vi "front_panel_v1.vi"() -> ()   [LabVIEW 2021]
uses:
  <vilib>/Platform/TimedLoop/XDataNode/timing_clust.ctl
  <vilib>/Platform/TimedLoop/XDataNode/nitl_modes.ctl
  <vilib>/Platform/TimedLoop/XDataNode/wakeup.ctl
  Global 1.vi
  <vilib>/platform/TimedLoop/XDataNode/XDataNode.xnode
  <vilib>/Platform/TimedLoop/XDataNode/XDNodeRunTimeDep.lvlib
panel:
  in  "Glove Address":string
  in  "Robotic Hand Address":string="192.168.4.93"
  out "Thumb 3":dbl
  out "Index Finger 2":dbl
  out "Middle Finger3":dbl
  out "Ring Finger 3":dbl
  out "Pinky Finger 2":dbl
  out "Simulation Connected":bool
  in  "Stop":bool
  in  "Stop Testing 2":bool
  out "Hand Status":bool
  out "Glove Status":bool
  in  "Stop Execution":bool
  in  "?":T1(tab)=enum."General Testing"
  out "Pinky Calibration":bool
  out "Ring Finger Calibration":bool
  out "Middle Finger Calibration":bool
  out "Index Calibration":bool
  out "Thumb Calibration":bool
  out "Glove SIgnal":dbl[](array[numeric])
  out "Waveform Chart":T2(graph)
  in  "Stop Testing":bool
  out "Output From Knob":string
  in  "Pinky":dbl(slide)
  in  "Ring Finger":dbl(slide)
  in  "Index":dbl(slide)
  in  "Middle Finger":dbl(slide)=85.0
  in  "Thumb":dbl(slide)=90.0
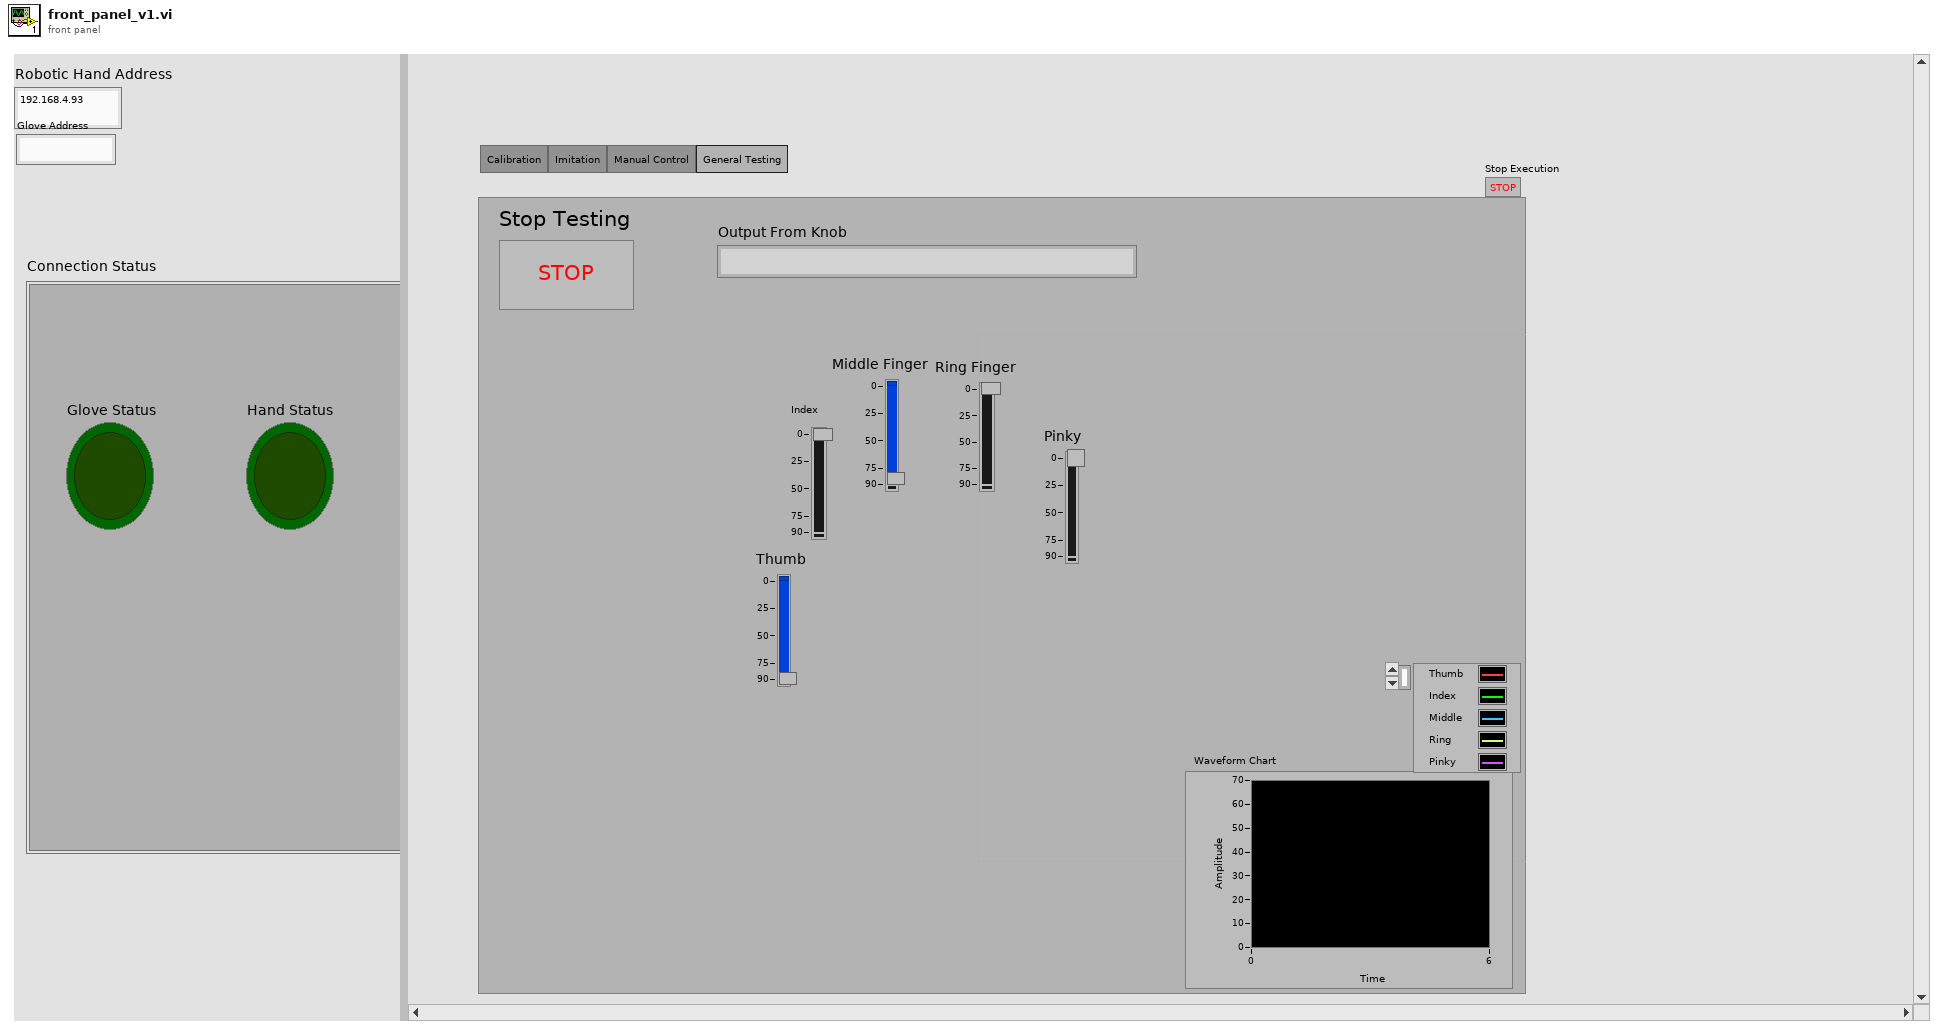
[diagram p1: front panel]
types:
  T1 = enum32{"Calibration", "Imitation", "Manual Control", "General Testing"}
  T2 = cluster{"[0]":dbl, "[1]":dbl, "[2]":dbl, "[3]":dbl, "[4]":dbl, "[5]":dbl, "[6]":dbl, "[7]":dbl, "[8]":dbl}
  T3 = cluster{"Clients":refnum<k5>[], "Listener":refnum<k5>}
  T4 = enum16{"Initialize", "Status Check", "Send Data", "Stop"}
  T5 = enum16{"Standard", "Buffered", "CRLF", "Immediate"}
  T6 = typedef "XDNodeRunTimeDep.lvlib/timing_clust.ctl" = cluster{"Expected End [f-1]":u64, "Actual End [f-1]":u64, "Finished Late? [f-1]":bool, "Expected End [i-1]":u64, "Actual End [i-1]":u64, "Finished Late? [i-1]":bool, "Expected Start [i]":u64, "Actual Start [i]":u64, "Expected Start [f]":u64, "Actual Start [f]":u64, "Source Name":string, "Structure Name":string, "Period":i64, "Deadline":i64, "Offset":i64, "Start":i64, "Priority":i32, "Timeout":i32, "Mode":T7, "Wakeup Reason":T8, "Error":errorcluster, "Source Type":string, "Secondary Source Type":string, "Global End Time":u64, "Global Start Time":u64, "Frame Duration":u64, "Iteration Duration":u64, "Assigned CPU":i32, "I/O Scan Engine Mode":u32}
  T7 = typedef "XDNodeRunTimeDep.lvlib/nitl_modes.ctl" = enum32{"No Change", "Process missed periods, maintain original phase", "Discard missed periods, maintain original phase", "Process missed periods, ignore original phase", "Discard missed periods, ignore original phase"}
  T8 = typedef "XDNodeRunTimeDep.lvlib/wakeup.ctl" = enum32{"Normal", "Aborted", "Asynchronous wakeup", "Timing source error", "Timed loop error", "Timeout"}
  T9 = cluster{"Glove output RT[0]":dbl, "Glove output RT[1]":dbl, "Glove output RT[2]":dbl, "Glove output RT[3]":dbl, "Glove output RT[4]":dbl, "Glove output RT[5]":dbl, "Glove output RT[6]":dbl, "Glove output RT[7]":dbl, "Glove output RT[8]":dbl}
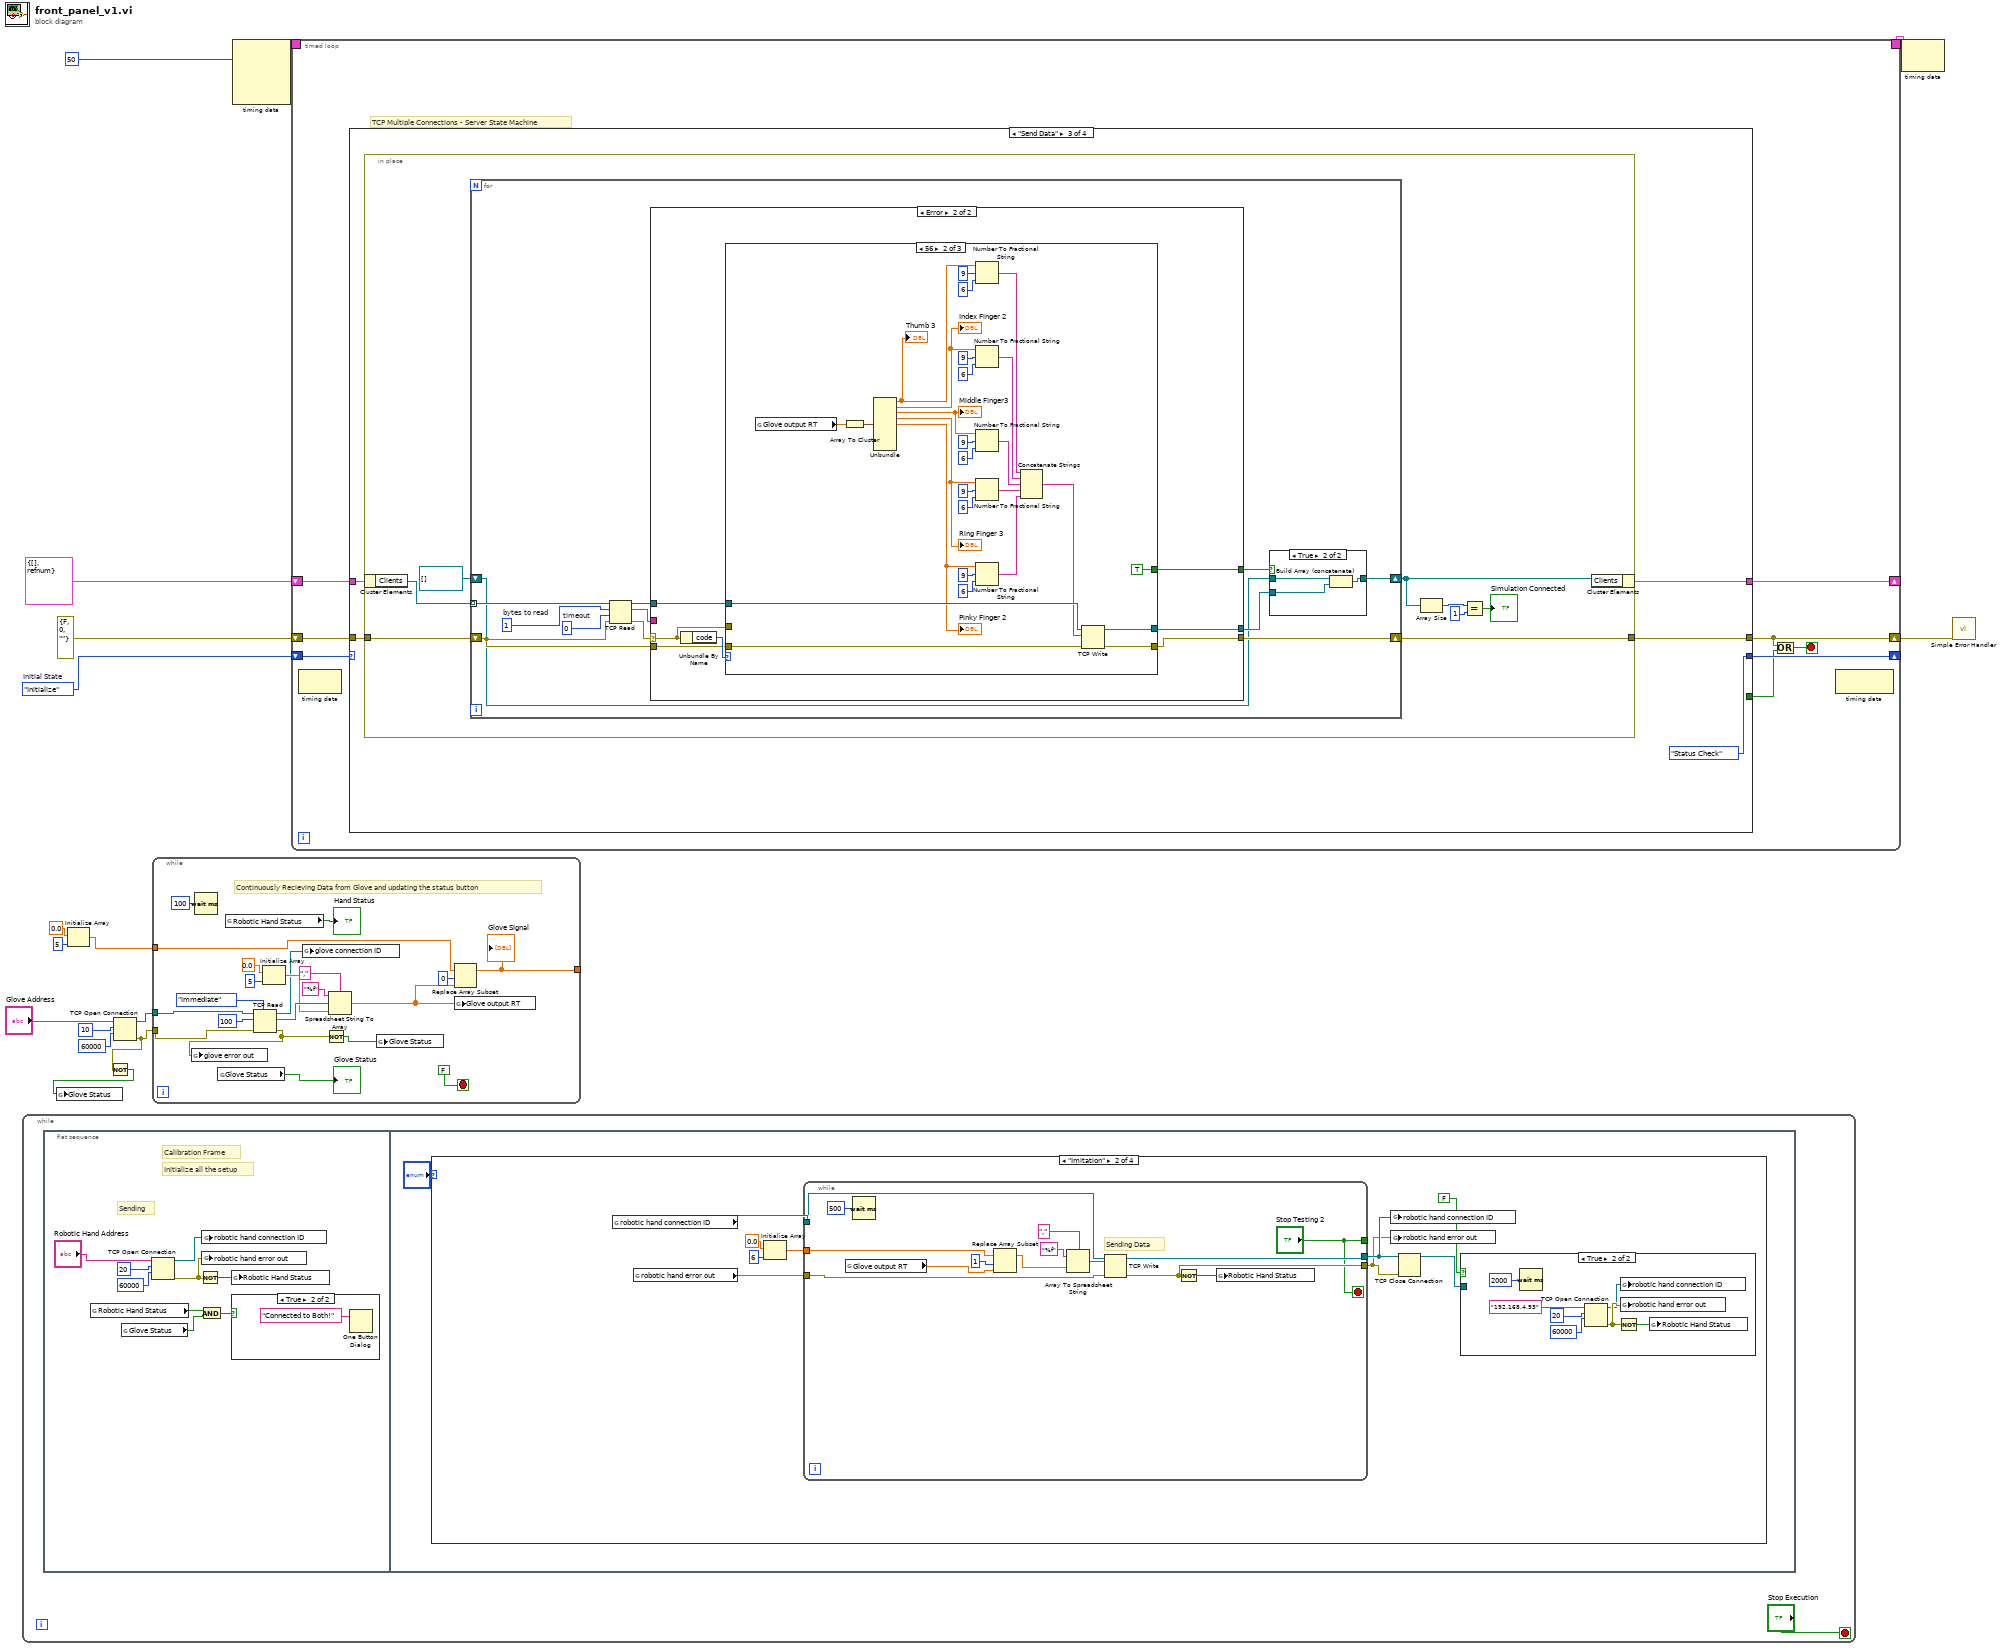
[diagram p0: block diagram]
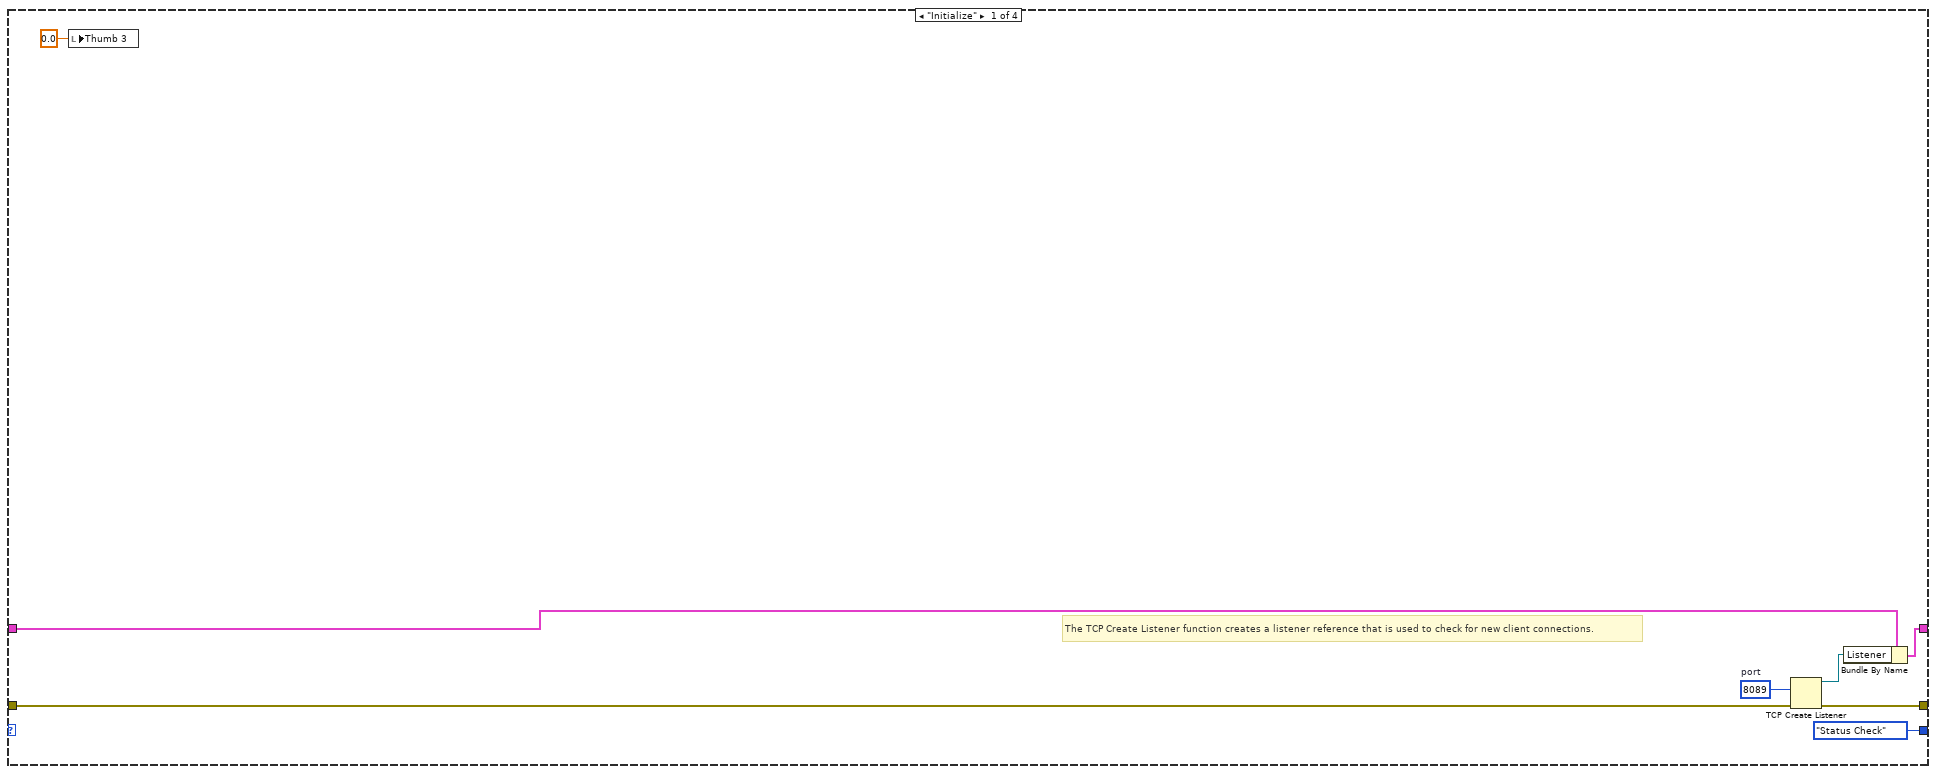
[diagram p2: hidden frame]
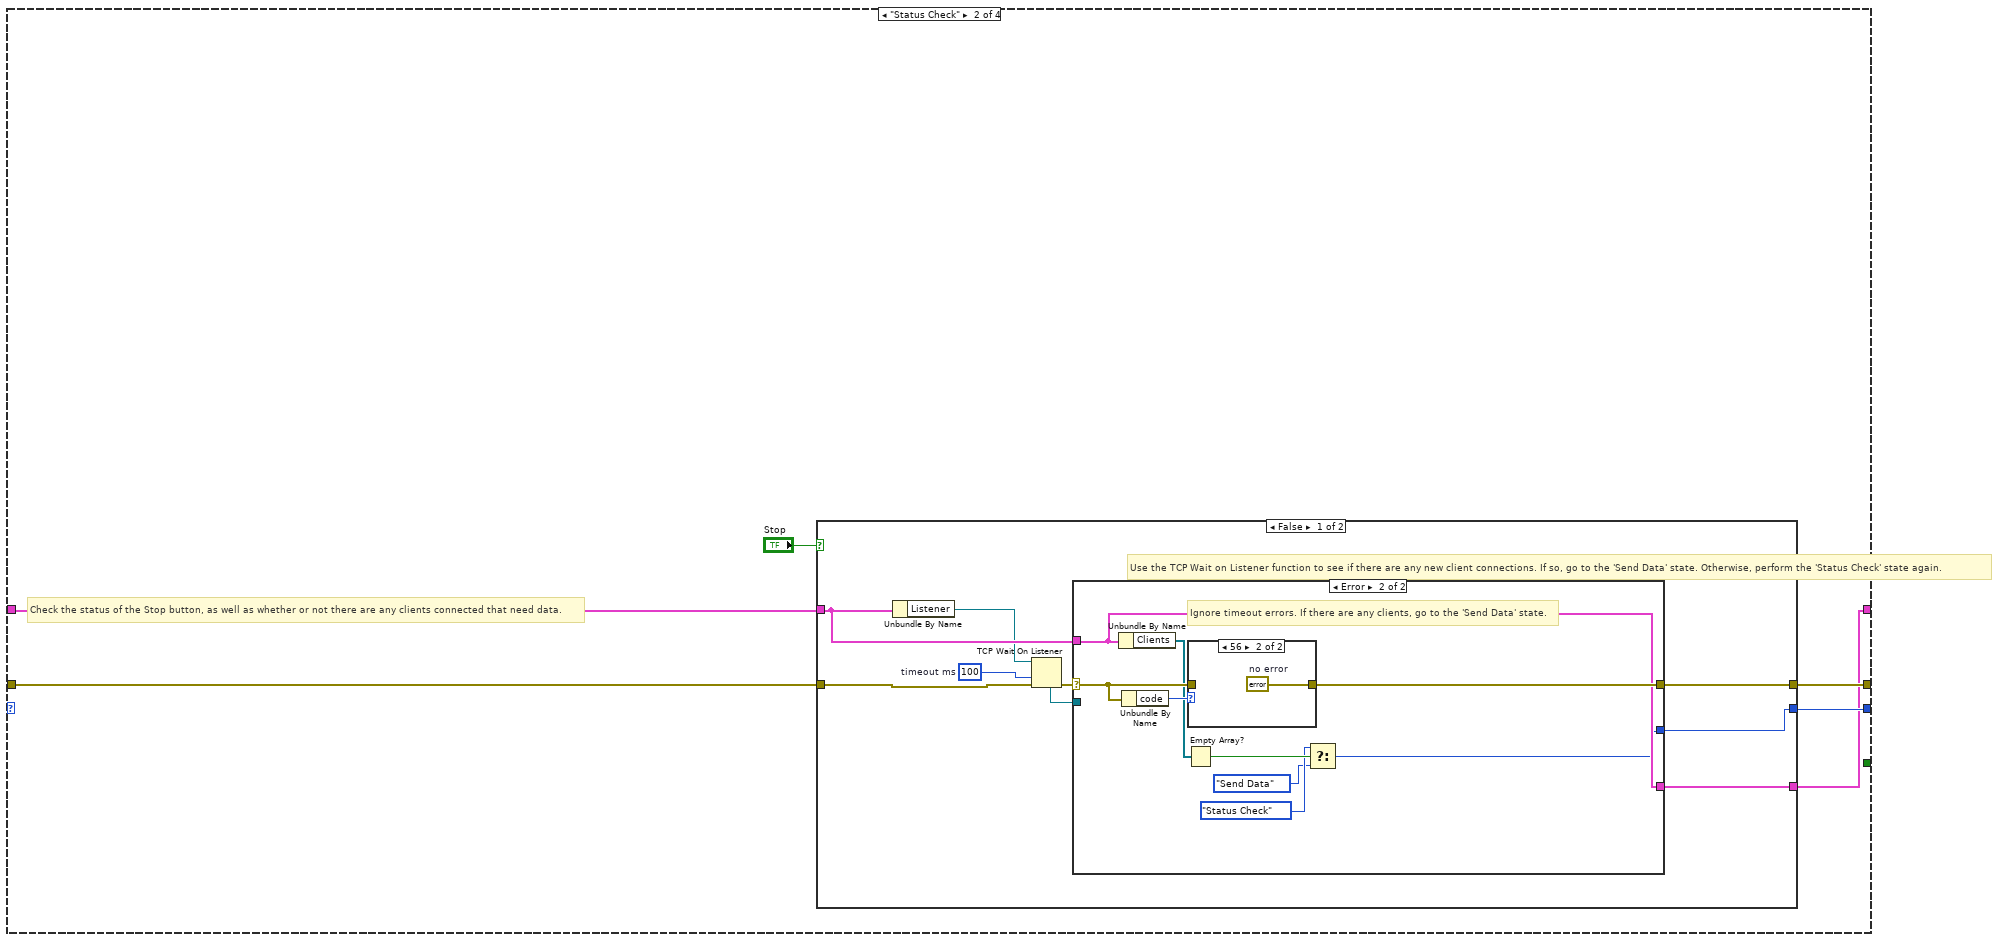
[diagram p3: hidden frame]
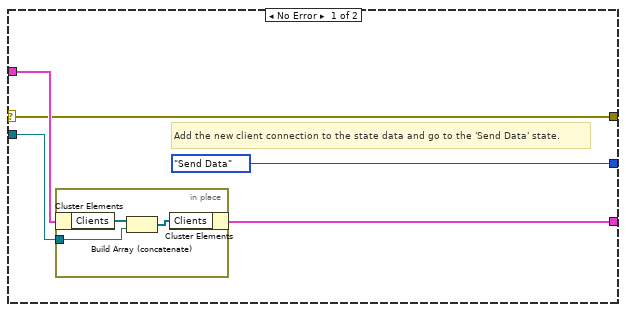
[diagram p4: hidden frame]
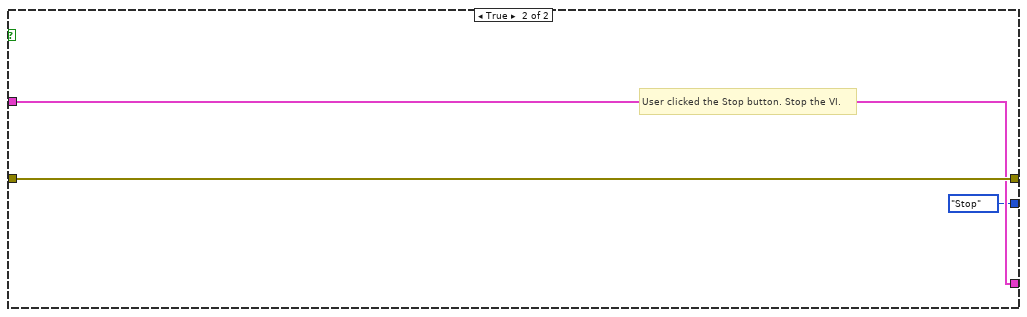
[diagram p6: hidden frame]
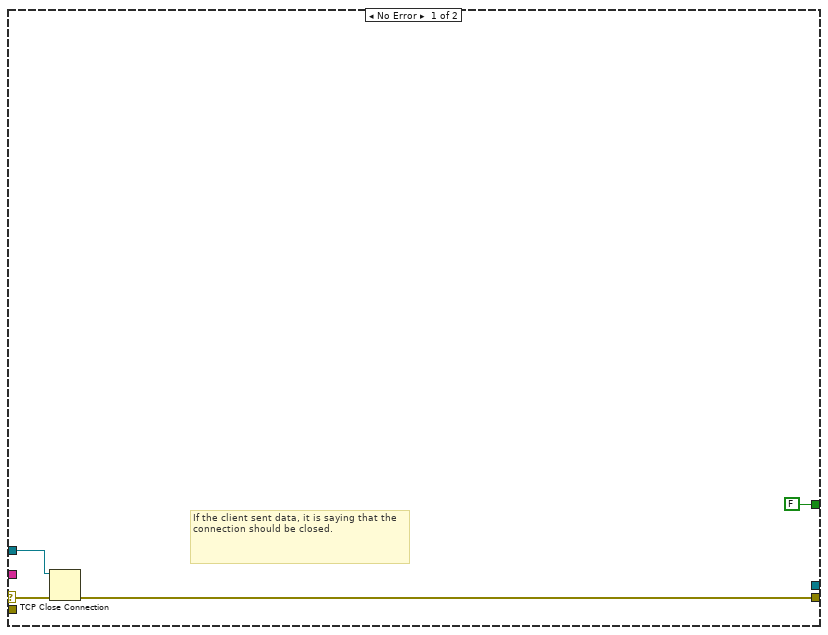
[diagram p8: hidden frame]
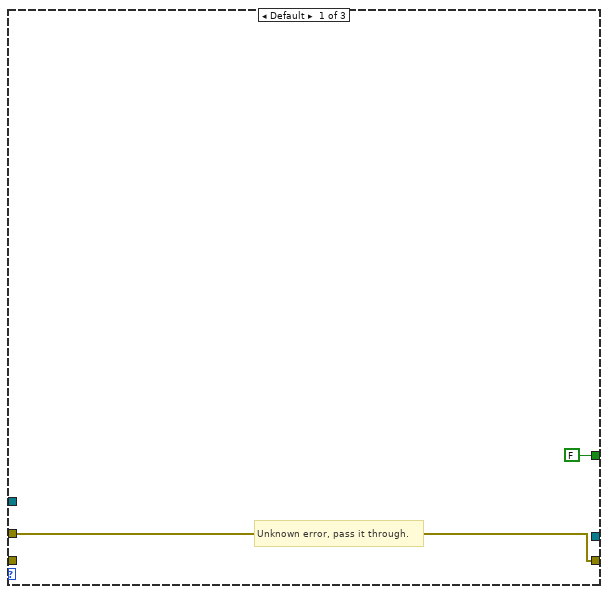
[diagram p9: hidden frame]
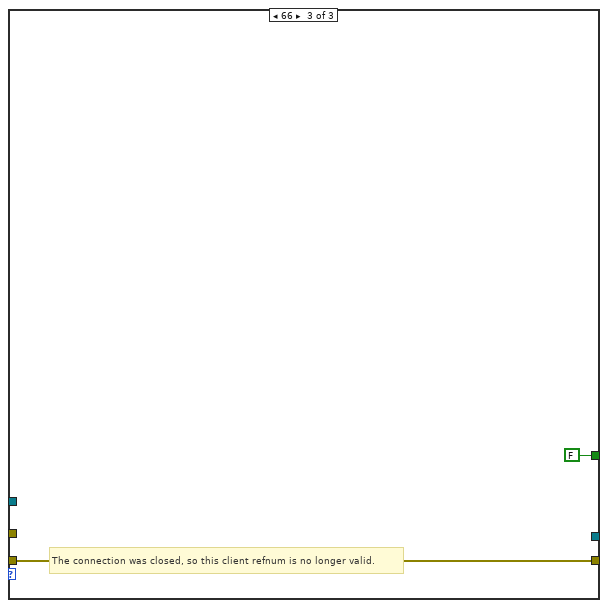
[diagram p10: hidden frame]
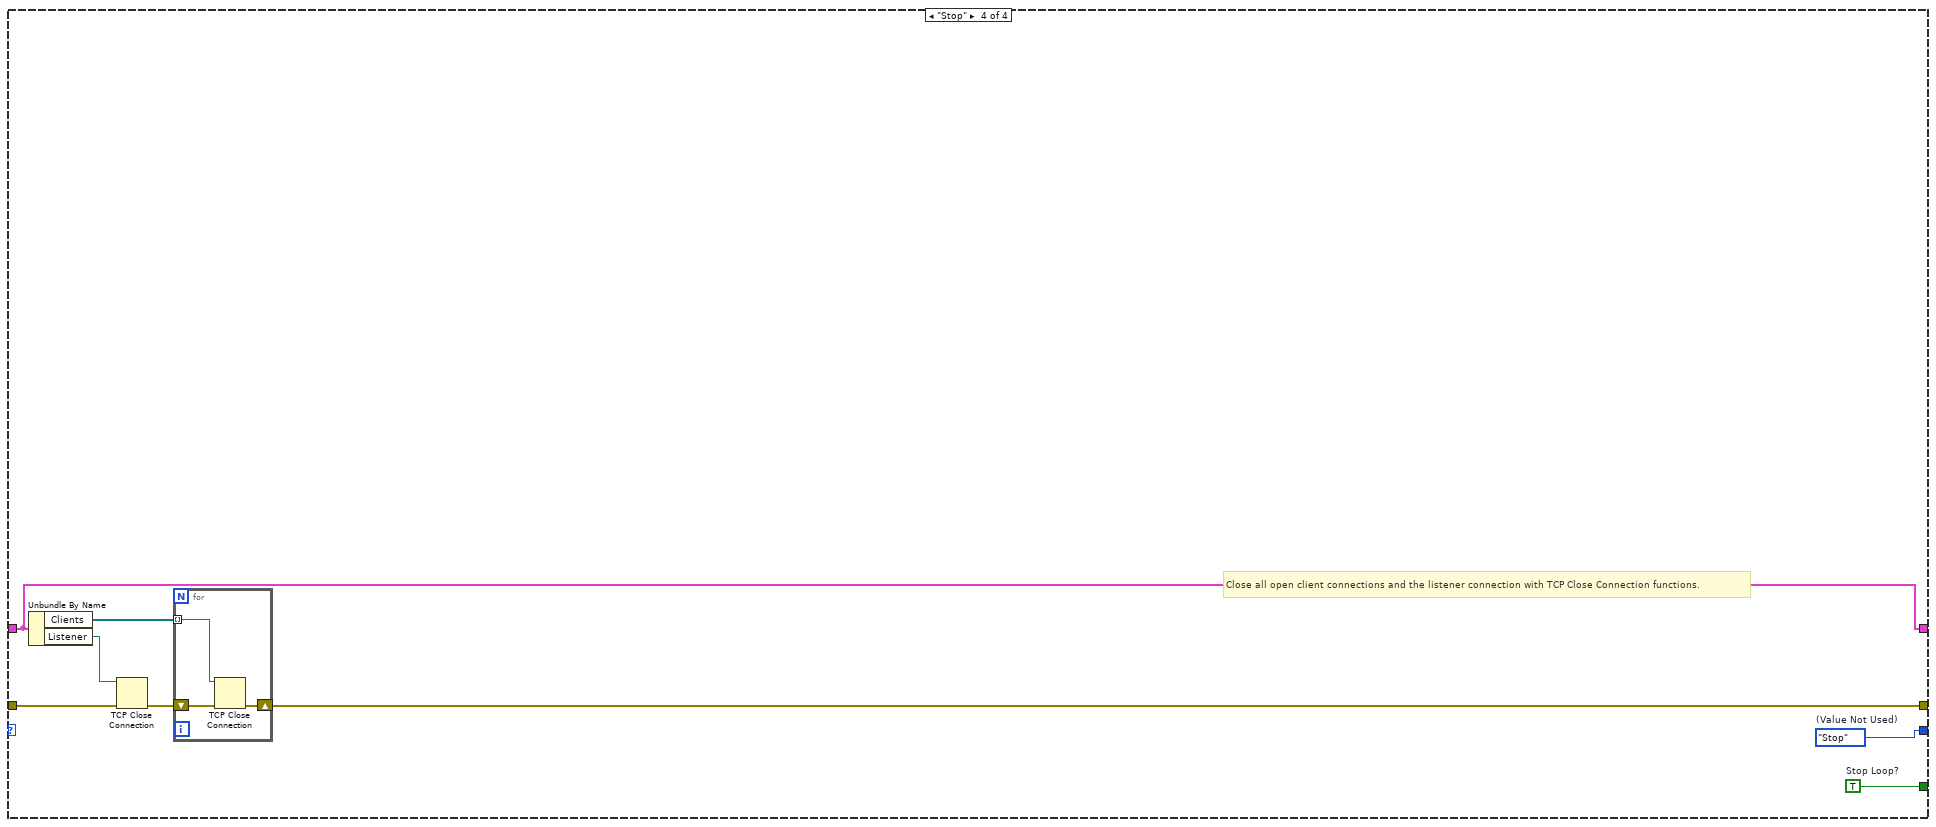
[diagram p11: hidden frame]
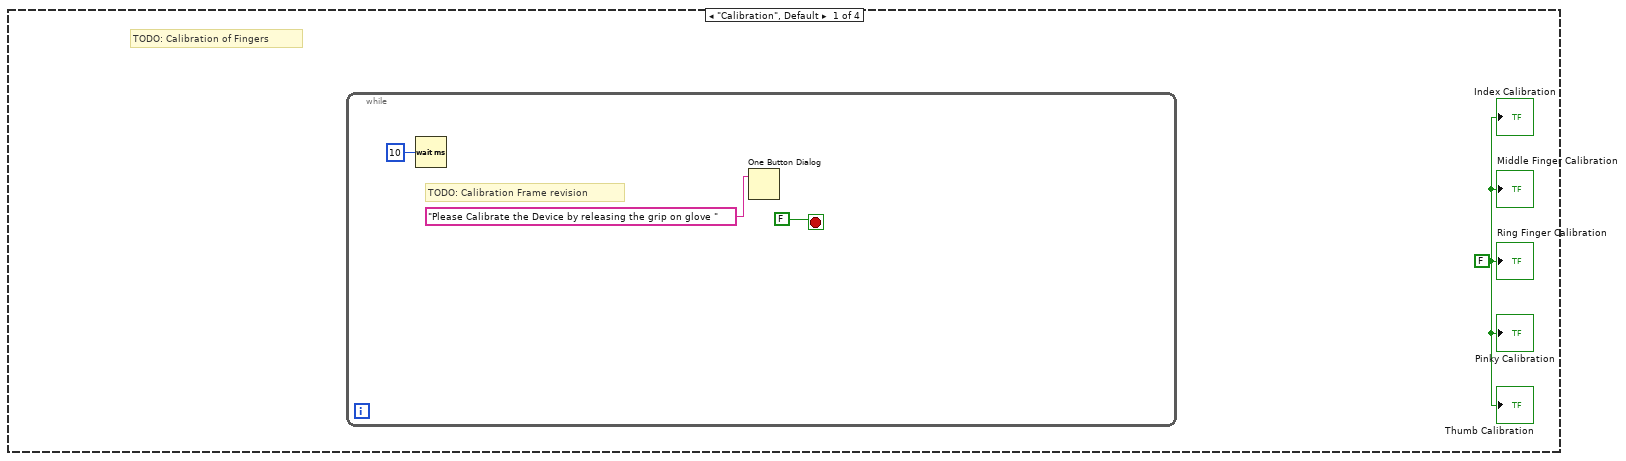
[diagram p13: hidden frame]
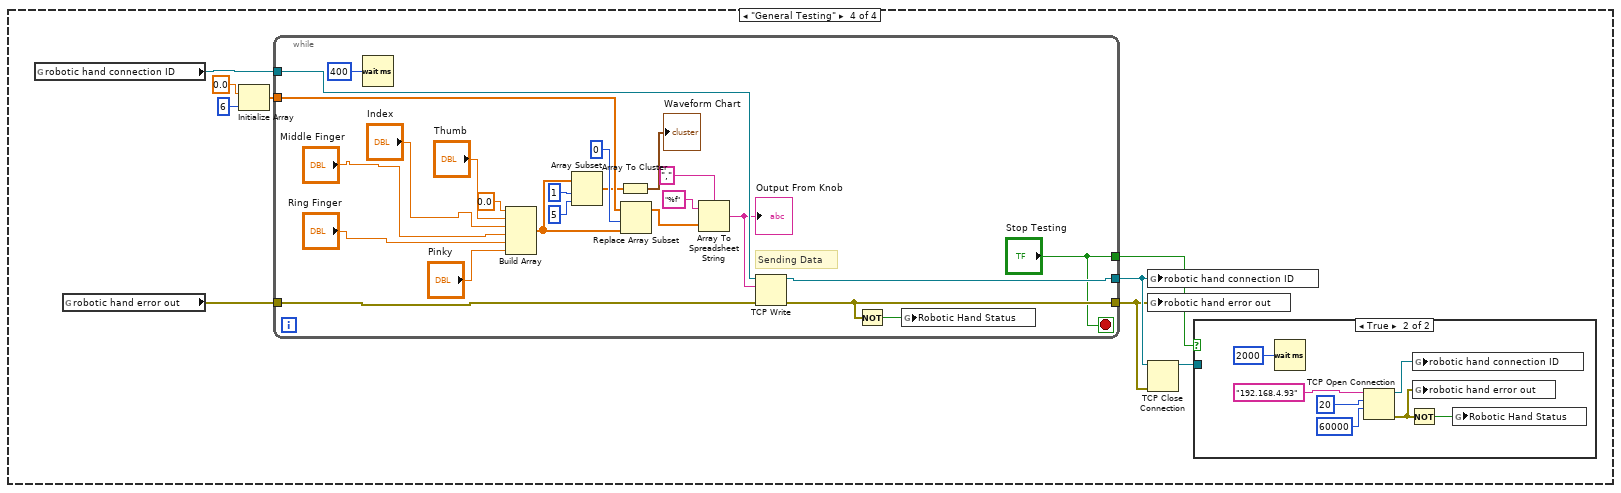
[diagram p16: hidden frame]
diagram:
  w16 = T4."Initialize"  # Initial State
  n1 = while {
    stop <- "Stop Execution" stop-if-true
    n2 = flat-sequence {
      frame #0 {
        # "Sending"
        # "Initialize all the setup"
        # "Calibration Frame"
        n3 = global read "Global 1.vi" "Robotic Hand Status"() -> (w24:bool)
        n4 = global read "Global 1.vi" "Glove Status"() -> (w25:bool)
        n5 = TCP Open Connection(address="Robotic Hand Address", remote port or service name=u16 20, timeout ms (60000)=60000) -> (connection ID=w21:refnum<k5>, error out=w22:errorcluster)  [unwired: 2 in]
        n6 = Not(x=w22) -> (.not. x?=w23:bool)
        n7 = And(x=w24, y=w25) -> (x .and. y?=w26:bool)
        n8 = global write "Global 1.vi" "robotic hand connection ID"(w21) -> ()
        n9 = global write "Global 1.vi" "robotic hand error out"(w22) -> ()
        n10 = global write "Global 1.vi" "Robotic Hand Status"(w23) -> ()
        n11 = case shown="True" w26 {
          frame False {
          }
          frame True {
            n12 = One Button Dialog(message="Connected to Both!") -> ()  [unwired: 1 in, 1 out]
          }
        }
      }
      frame #1 {
        n13 = case shown="\"Imitation\"" "?" {
          frame "Calibration", Default {
            w29 = FALSE ("Index Calibration")
            # "TODO: Calibration of Fingers"
            n14 = while {
              stop <- FALSE stop-if-true
              # "TODO: Calibration Frame revision"
              n15 = Wait (ms)(milliseconds to wait=u32 10) -> ()  [unwired: 1 out]
              n16 = One Button Dialog(message="Please Calibrate the Device by releasing the grip on glove ") -> ()  [unwired: 1 in, 1 out]
            }
            "Thumb Calibration" <- w29
            "Index Calibration" <- w29
            "Middle Finger Calibration" <- w29
            "Ring Finger Calibration" <- w29
            "Pinky Calibration" <- w29
          }
          frame "Imitation" {
            n17 = global read "Global 1.vi" "robotic hand connection ID"() -> (w39:refnum<k5>)
            n18 = global read "Global 1.vi" "robotic hand error out"() -> (w38:errorcluster)
            n19 = Initialize Array(0.0 ("element"), 6 ("dimension size")) -> (w40:dbl[])
            n20 = while {
              tunnel: [w62] -> w37
              tunnel: w39 -> [w61]
              tunnel: w38 -> [w59]
              tunnel: [w52] -> w36
              tunnel: w40 -> [w50]
              tunnel: ["Stop Testing 2"] -> _
              stop <- "Stop Testing 2" stop-if-true
              # "Sending Data"
              n21 = global read "Global 1.vi" "Glove output RT"() -> (w49:dbl[])
              n22 = Wait (ms)(milliseconds to wait=u32 500) -> ()  [unwired: 1 out]
              n23 = Replace Array Subset(array=w50, new element=w49, index=1) -> (w56:dbl[])
              n24 = Array To Spreadsheet String(delimiter (Tab)=",", array=w56, 3:"%f" ("format string")) -> (spreadsheet string=w54:string)
              n25 = TCP Write(connection ID=w61, data in=w54, error in (no error)=w59) -> (connection ID out=w62:refnum<k5>, error out=w52:errorcluster)  [unwired: 1 in, 1 out]
              n26 = Not(x=w52) -> (.not. x?=w53:bool)
              n27 = global write "Global 1.vi" "Robotic Hand Status"(w53) -> ()
            }
            n28 = global write "Global 1.vi" "robotic hand connection ID"(w37) -> ()
            n29 = global write "Global 1.vi" "robotic hand error out"(w36) -> ()
            n30 = TCP Close Connection(connection ID=w37, error in (no error)=w36) -> (connection ID out=w35:refnum<k5>)  [unwired: 1 in, 1 out]
            n31 = case shown="True" FALSE {
              tunnel: w35 -> [_ _]
              frame False {
              }
              frame True {
                n32 = Wait (ms)(milliseconds to wait=u32 2000) -> ()  [unwired: 1 out]
                n33 = TCP Open Connection(address="192.168.4.93", remote port or service name=u16 20, timeout ms (60000)=60000) -> (connection ID=w46:refnum<k5>, error out=w47:errorcluster)  [unwired: 2 in]
                n34 = Not(x=w47) -> (.not. x?=w48:bool)
                n35 = global write "Global 1.vi" "robotic hand connection ID"(w46) -> ()
                n36 = global write "Global 1.vi" "robotic hand error out"(w47) -> ()
                n37 = global write "Global 1.vi" "Robotic Hand Status"(w48) -> ()
              }
            }
          }
          frame "Manual Control" {
          }
          frame "General Testing" {
            n38 = global read "Global 1.vi" "robotic hand connection ID"() -> (w68:refnum<k5>)
            n39 = global read "Global 1.vi" "robotic hand error out"() -> (w67:errorcluster)
            n40 = Initialize Array(0.0 ("element"), 6 ("dimension size")) -> (w69:dbl[])
            n41 = while {
              tunnel: [w102] -> w66
              tunnel: w68 -> [w101]
              tunnel: w67 -> [w99]
              tunnel: [w91] -> w65
              tunnel: w69 -> [w93]
              tunnel: ["Stop Testing"] -> w64
              stop <- "Stop Testing" stop-if-true
              # "Sending Data"
              n42 = Wait (ms)(milliseconds to wait=u32 400) -> ()  [unwired: 1 out]
              n43 = Build Array(0.0 ("element"), "Thumb", "Index", "Middle Finger", "Ring Finger", "Pinky") -> (w87:dbl[])
              n44 = Array Subset(array=w87, index=1, length=5) -> (w86:dbl[])
              n45 = Array To Cluster(array=w86) -> (cluster=→"Waveform Chart":T2)
              n46 = Replace Array Subset(array=w93, new element=w87, index=0) -> (w96:dbl[])
              n47 = Array To Spreadsheet String(delimiter (Tab)=",", array=w96, 3:"%f" ("format string")) -> (spreadsheet string=w94:string)
              "Output From Knob" <- w94
              n48 = TCP Write(connection ID=w101, data in=w94, error in (no error)=w99) -> (connection ID out=w102:refnum<k5>, error out=w91:errorcluster)  [unwired: 1 in, 1 out]
              n49 = Not(x=w91) -> (.not. x?=w92:bool)
              n50 = global write "Global 1.vi" "Robotic Hand Status"(w92) -> ()
            }
            n51 = global write "Global 1.vi" "robotic hand connection ID"(w66) -> ()
            n52 = global write "Global 1.vi" "robotic hand error out"(w65) -> ()
            n53 = TCP Close Connection(connection ID=w66, error in (no error)=w65) -> (connection ID out=w63:refnum<k5>)  [unwired: 1 in, 1 out]
            n54 = case shown="True" w64 {
              tunnel: w63 -> [_ _]
              frame False {
              }
              frame True {
                n55 = Wait (ms)(milliseconds to wait=u32 2000) -> ()  [unwired: 1 out]
                n56 = TCP Open Connection(address="192.168.4.93", remote port or service name=u16 20, timeout ms (60000)=60000) -> (connection ID=w76:refnum<k5>, error out=w77:errorcluster)  [unwired: 2 in]
                n57 = Not(x=w77) -> (.not. x?=w78:bool)
                n58 = global write "Global 1.vi" "robotic hand connection ID"(w76) -> ()
                n59 = global write "Global 1.vi" "robotic hand error out"(w77) -> ()
                n60 = global write "Global 1.vi" "Robotic Hand Status"(w78) -> ()
              }
            }
          }
        }
      }
    }
  }
  n61 = Initialize Array(0.0 ("element"), 5 ("dimension size")) -> (w3:dbl[])
  n62 = TCP Open Connection(address="Glove Address", remote port or service name=u16 10, timeout ms (60000)=60000) -> (connection ID=w8:refnum<k5>, error out=w9:errorcluster)  [unwired: 2 in]
  n63 = Not(x=w9) -> (.not. x?=w12:bool)
  n64 = global write "Global 1.vi" "Glove Status"(w12) -> ()
  n65 = while {
    tunnel: w8 -> [w110]
    tunnel: w9 -> [w109]
    tunnel: w3 -> [w104]
    tunnel: [w103] -> _
    stop <- FALSE stop-if-true
    # "Continuously Recieving Data from Glove and updating the status button"
    n66 = Wait (ms)(milliseconds to wait=u32 100) -> ()  [unwired: 1 out]
    n67 = global read "Global 1.vi" "Glove Status"() -> (→"Glove Status":bool)
    n68 = global read "Global 1.vi" "Robotic Hand Status"() -> (→"Hand Status":bool)
    n69 = TCP Read(connection ID=w110, bytes to read=100, error in (no error)=w109, 7:T5."Immediate" ("mode (standard)")) -> (connection ID out=w111:refnum<k5>, data out=w117:string, error out=w107:errorcluster)  [unwired: 1 in]
    n70 = global write "Global 1.vi" "glove error out"(w107) -> ()
    n71 = Initialize Array(0.0 ("element"), 5 ("dimension size")) -> (w116:dbl[])
    n72 = global write "Global 1.vi" "glove connection ID"(w111) -> ()
    n73 = Not(x=w107) -> (.not. x?=w108:bool)
    n74 = Spreadsheet String To Array(delimiter (Tab)=",", format string="%f", spreadsheet string=w117, array type (2D Dbl)=w116) -> (array=w106:dbl[])
    n75 = global write "Global 1.vi" "Glove Status"(w108) -> ()
    n76 = Replace Array Subset(array=w104, new element=w106, index=0) -> (w103:dbl[])
    "Glove SIgnal" <- w103
    n77 = global write "Global 1.vi" "Glove output RT"(w106) -> ()
  }
  n78 = node-c288(i64 50 ("Period")) -> (w7:T6)  [unwired: 3 in]
  n79 = timed-loop {
    shift-right: [w130] -> _
    shift-left: w16 -> [w131]
    shift-right: [w128] -> _
    shift-left: T3 {"Clients"=[], "Listener"=refnum} ("Data") -> [w129]
    shift-right: [w124] -> w14
    shift-left: errorcluster {"status"=FALSE, "code"=0, "source"=""} ("error constant") -> [w127]
    timing: w7 -> [_]
    timing-out: [_] -> w6
    stop <- w125 stop-if-true
    # "TCP Multiple Connections - Server State Machine"
    n80 = node-c288() -> ()  [unwired: 1 in, 1 out]
    n81 = case shown="\"Send Data\"" w131 {
      tunnel: [T4."Status Check" ("States") w147 T4."Status Check" ("States") w251] -> w130
      tunnel: [_ _ _ w258] -> w126
      tunnel: w129 -> [w139 w143 w181 w257]
      tunnel: [w138 w142 w180 w257] -> w128
      tunnel: w127 -> [w141 w146 w183 w256]
      tunnel: [w140 w145 w182 w254] -> w124
      frame "Initialize" {
        w136 = u16 8089  # port
        # "The TCP Create Listener function creates a listener reference that is used to check for new client connections."
        n82 = local write "Thumb 3"(0.0 ("Current Data")) -> ()
        n83 = TCP Create Listener(8:w141, 10:w136) -> (0:w140:errorcluster, 3:w137:refnum<k5>)  [unwired: 4 out]
        n84 = Bundle By Name(cluster=w139, "Listener"=w137) -> (w138:T3)
      }
      frame "Status Check" {
        # "Check the status of the Stop button, as well as whether or not there are any clients connected that need data."
        n85 = case shown="False" "Stop" {
          tunnel: [w156 T4."Stop" ("States")] -> w147
          tunnel: w146 -> [w155 w178]
          tunnel: [w148 w178] -> w145
          tunnel: w143 -> [w151 w177]
          tunnel: [w150 w177] -> w142
          frame False {
            w154 = 100  # timeout ms
            # "Use the TCP Wait on Listener function to see if there are any new client connections. If so, go to the 'Send Data' state. Otherwise, perform the 'Status Check' state again."
            n86 = Unbundle By Name(w151) -> ("Listener"=w149:refnum<k5>)
            n87 = TCP Wait On Listener(8:w155, 9:w154, 11:w149) -> (0:w153:errorcluster, 4:w152:refnum<k5>)  [unwired: 4 out]
            n88 = case shown="Error" w153 {
              selector: w153 -> [w159 w173]
              tunnel: [T4."Send Data" ("States") w167] -> w156
              tunnel: w152 -> [w160 _]
              tunnel: w151 -> [w161 w170]
              tunnel: [w158 w170] -> w150
              tunnel: [w159 w171] -> w148
              frame No Error {
                # "Add the new client connection to the state data and go to the 'Send Data' state."
                n89 = in-place {
                  in-place-border: w160 -> [w162]
                  n90 = in-place-cluster #1(w161) -> ("Clients"=w164:refnum<k5>[])
                  n91 = Build Array (concatenate)(w164, w162) -> (w163:refnum<k5>[])
                  n92 = in-place-cluster #1("Clients"=w163) -> (w158:T3)
                }
              }
              frame Error {
                # "Ignore timeout errors. If there are any clients, go to the 'Send Data' state."
                n93 = Unbundle By Name(w170) -> ("Clients"=w169:refnum<k5>[])
                n94 = Unbundle By Name(w173) -> ("code"=w172:i32)
                n95 = Empty Array?(array=w169) -> (empty?=w168:bool)
                n96 = case shown="56" w172 {
                  tunnel: w173 -> [w174 _]
                  tunnel: [w174 w175] -> w171
                  frame Default {
                  }
                  frame 56 {
                    w175 = errorcluster {"status"=FALSE, "code"=0, "source"=""}  # no error
                  }
                }
                n97 = Select(t=T4."Status Check" ("States"), s=w168, f=T4."Send Data" ("States")) -> (s? t:f=w167:T4)
              }
            }
          }
          frame True {
            # "User clicked the Stop button. Stop the VI."
          }
        }
      }
      frame "Send Data" {
        n98 = in-place {
          in-place-border: w183 -> [w191]
          in-place-border: [w190] -> w182
          n99 = in-place-cluster #2(w181) -> ("Clients"=w189:refnum<k5>[])
          n100 = for {
            tunnel: w189 -> [w203] mode=indexing
            shift-right: [w195] -> w190
            shift-left: w191 -> [w194]
            shift-right: [w192] -> w188
            shift-left: refnum<k5>[] [] ("Array") -> [w193]
            w200 = 0  # timeout
            w201 = 1  # bytes to read
            n101 = TCP Read(connection ID=w203, bytes to read=w201, error in (no error)=w194, 9:w200) -> (connection ID out=w202:refnum<k5>, data out=w198:string, error out=w199:errorcluster)  [unwired: 1 out]
            n102 = case shown="Error" w199 {
              selector: w199 -> [w210 w217]
              tunnel: w202 -> [w211 w214]
              tunnel: w198 -> [_ _]
              tunnel: [_ w212] -> w197
              tunnel: [FALSE w213] -> w196
              tunnel: [w208 w216] -> w195
              tunnel: w194 -> [_ w215]
              frame No Error {
                # "If the client sent data, it is saying that the connection should be closed."
                # "If the client sent data, it is saying that the connection should be closed."
                n103 = TCP Close Connection(connection ID=w211, error in (no error)=w210) -> (error out=w208:errorcluster)  [unwired: 2 out]
              }
              frame Error {
                # "Ignore connection closed and timeout errors"
                n104 = Unbundle By Name(w217) -> ("code"=w218:i32)
                n105 = case shown="56" w218 {
                  tunnel: w217 -> [w220 _ _]
                  tunnel: [w220 w248 w250] -> w216
                  tunnel: w215 -> [_ w244 w250]
                  tunnel: w214 -> [_ w247 _]
                  tunnel: [FALSE TRUE FALSE] -> w213
                  tunnel: [_ w246 _] -> w212
                  frame Default {
                    # "Unknown error, pass it through."
                  }
                  frame 56 {
                    n106 = global read "Global 1.vi" "Glove output RT"() -> (w227:dbl[])
                    n107 = Array To Cluster(array=w227) -> (cluster=w226:T9)
                    n108 = Unbundle(w226) -> ("Glove output RT[0]"=w223:dbl, "Glove output RT[1]"=w224:dbl, "Glove output RT[2]"=w225:dbl, "Glove output RT[3]"=w222:dbl, "Glove output RT[4]"=w221:dbl)  [unwired: 4 out]
                    "Thumb 3" <- w223
                    "Index Finger 2" <- w224
                    "Middle Finger3" <- w225
                    "Ring Finger 3" <- w222
                    "Pinky Finger 2" <- w221
                    n109 = Number To Fractional String(number=w223, width (-)=i16 9, precision (6)=i16 6) -> (F-format string=w242:string)  [unwired: 1 in]
                    n110 = Number To Fractional String(number=w224, width (-)=i16 9, precision (6)=i16 6) -> (F-format string=w241:string)  [unwired: 1 in]
                    n111 = Number To Fractional String(number=w225, width (-)=i16 9, precision (6)=i16 6) -> (F-format string=w240:string)  [unwired: 1 in]
                    n112 = Number To Fractional String(number=w222, width (-)=i16 9, precision (6)=i16 6) -> (F-format string=w239:string)  [unwired: 1 in]
                    n113 = Number To Fractional String(number=w221, width (-)=i16 9, precision (6)=i16 6) -> (F-format string=w238:string)  [unwired: 1 in]
                    n114 = Concatenate Strings(w242, w241, w240, w239, w238) -> (w243:string)
                    n115 = TCP Write(connection ID=w247, data in=w243, error in (no error)=w244) -> (connection ID out=w246:refnum<k5>, error out=w248:errorcluster)  [unwired: 2 out]
                  }
                  frame 66 {
                    # "The connection was closed, so this client refnum is no longer valid."
                  }
                }
              }
            }
            n116 = case shown="True" w196 {
              tunnel: w193 -> [w204 w206]
              tunnel: w197 -> [_ w205]
              tunnel: [w204 w207] -> w192
              frame False {
              }
              frame True {
                n117 = Build Array (concatenate)(w206, w205) -> (w207:refnum<k5>[])
              }
            }
          }
          n118 = Array Size(array=w188) -> (size(s)=w186:i32)
          n119 = Equal?(x=w186, y=1) -> (x = y?=→"Simulation Connected":bool)
          n120 = in-place-cluster #2("Clients"=w188) -> (w180:T3)
        }
      }
      frame "Stop" {
        w251 = T4."Stop"  # (Value Not Used)
        w258 = TRUE  # Stop Loop?
        # "Close all open client connections and the listener connection with TCP Close Connection functions."
        n121 = Unbundle By Name(w257) -> ("Clients"=w255:refnum<k5>[], "Listener"=w252:refnum<k5>)
        n122 = TCP Close Connection(connection ID=w252, error in (no error)=w256) -> (error out=w253:errorcluster)  [unwired: 1 in, 1 out]
        n123 = for {
          shift-right: [w260] -> w254
          shift-left: w253 -> [w261]
          tunnel: w255 -> [w259] mode=indexing
          n124 = TCP Close Connection(connection ID=w259, error in (no error)=w261) -> (error out=w260:errorcluster)  [unwired: 1 in, 1 out]
        }
      }
    }
    n125 = Or(x=w124, y=w126) -> (x .or. y?=w125:bool)
    n126 = node-c288() -> ()  [unwired: 1 in, 1 out]
  }
  n127 = node-c288(w6) -> ()  [unwired: 1 out]
  n128 = call <vilib>:"Simple Error Handler.vi"("error in (no error)"=w14) -> ()  [unwired: 4 in, 5 out]
